vi "EchoSpacing.vi"() -> ()   [LabVIEW 2016]
uses:
  <vilib>/Analysis/3filter.llb/Filter Passband Type.ctl
  <vilib>/measure/NI_MABase.lvlib
  <vilib>/Analysis/NI_AALBase.lvlib
  <vilib>/measure/NI_MAPro.lvlib
panel:
  in  "Vertical Shift":dbl format="%#_13g"
  out "output waveform":waveform(dbl)(graph)
  out "Waveforms":waveform(dbl)[](graph)=[{"t0"=timestamp(0 s since 1904-01-01), "dt"=1e-06, "Y"=array[1000000 elements]}, {"t0"=timestamp(0 s since 1904-01-01), "dt"=1e-06, "Y"=array[1000000 elements]}]
  out "Waveform":waveform(dbl)(graph)={"t0"=timestamp(0 s since 1904-01-01), "dt"=1e-06, "Y"=array[1000000 elements]}
  in  "threshold":dbl format="%0.2f"
  in  "width":i32=3 min=3
  in  "low cutoff freq: fl":dbl=10.0 format="%0.4f"
  out "error":i32
  in  "order":i32=3
  out "total time":u32=122
  in  "frequency":dbl=40.0 format="%0.2p"
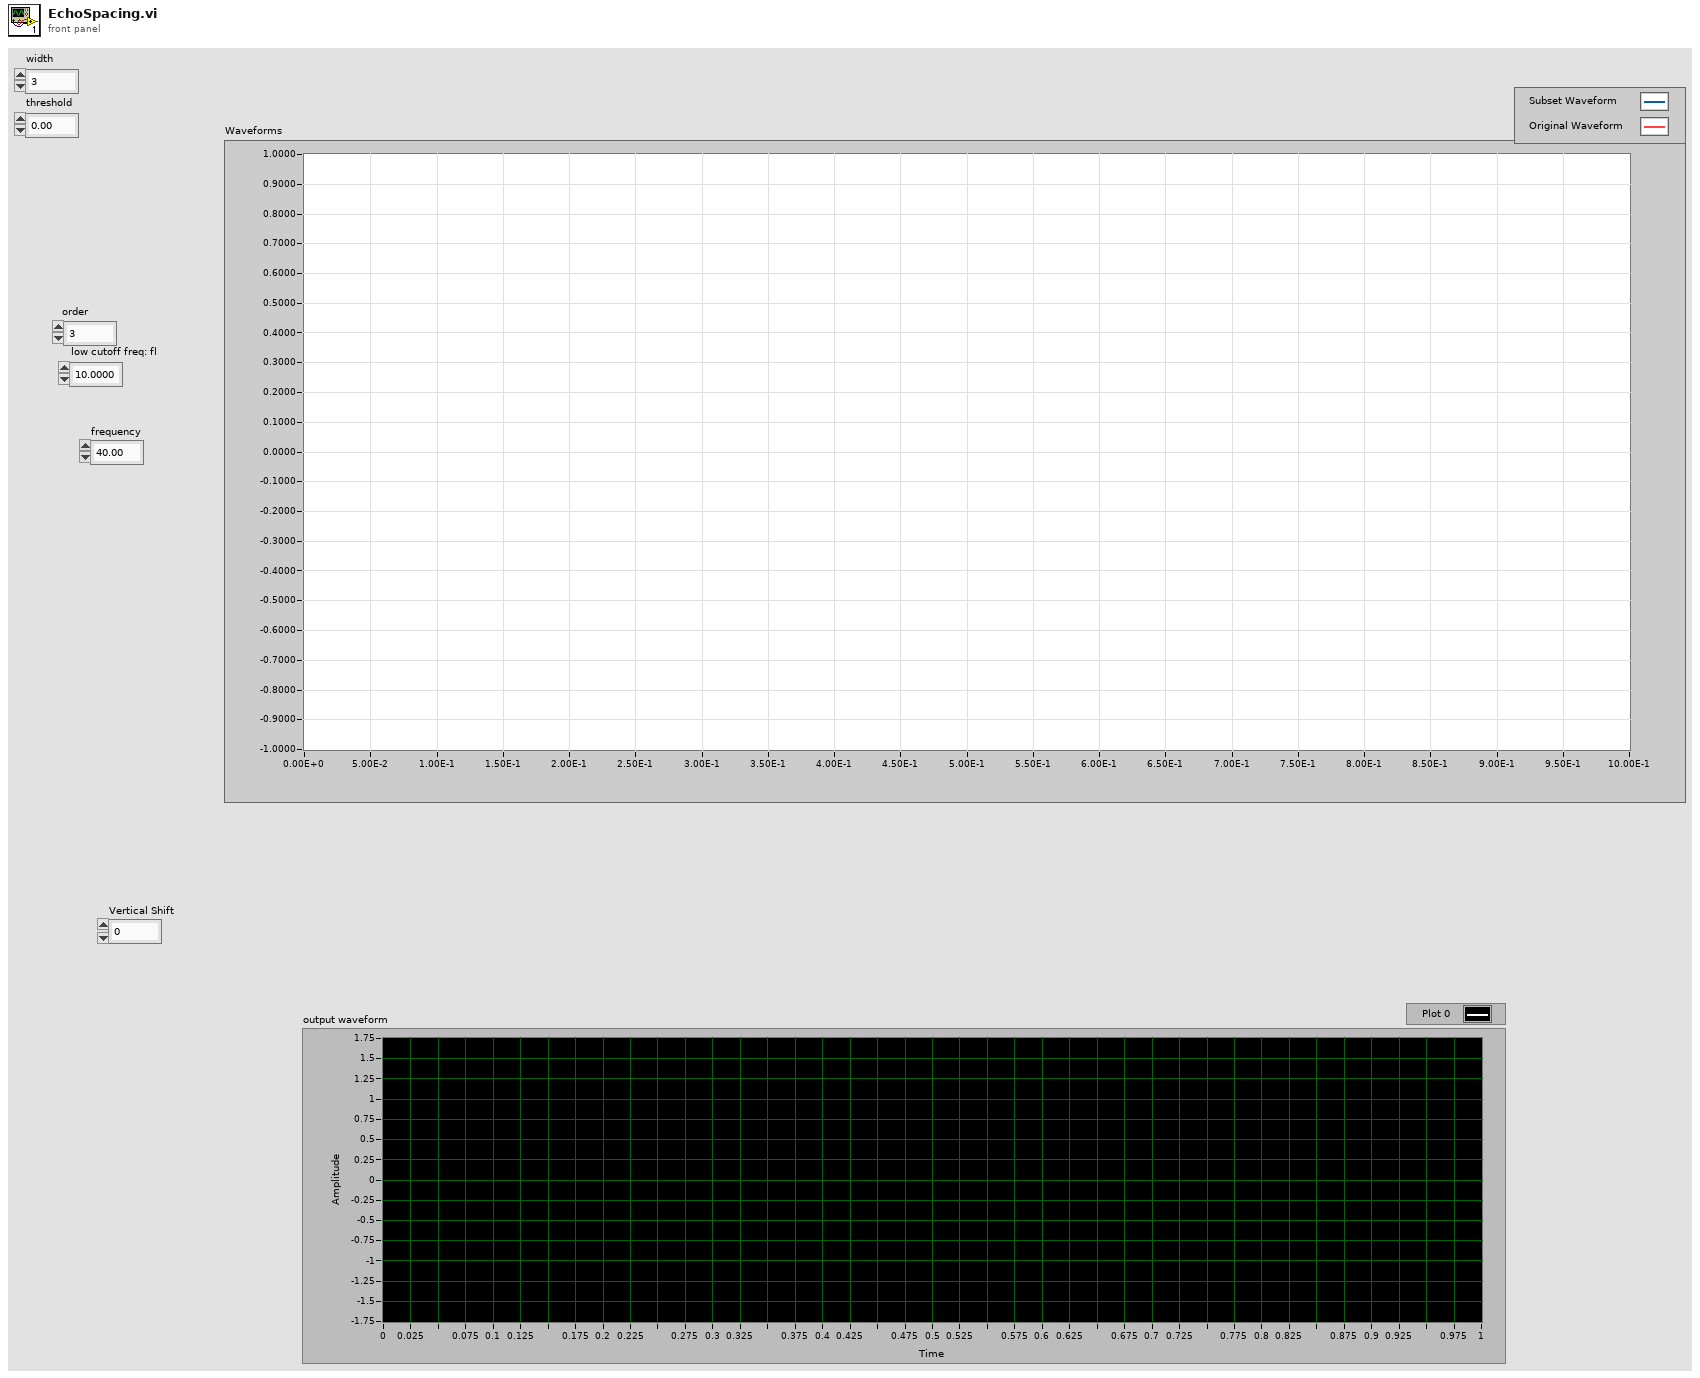
[diagram p1: front panel]
types:
  T1 = typedef "NI_AALBase.lvlib/Filter Passband Type.ctl" = enum32{"Lowpass", "Highpass", "Bandpass", "Bandstop"}
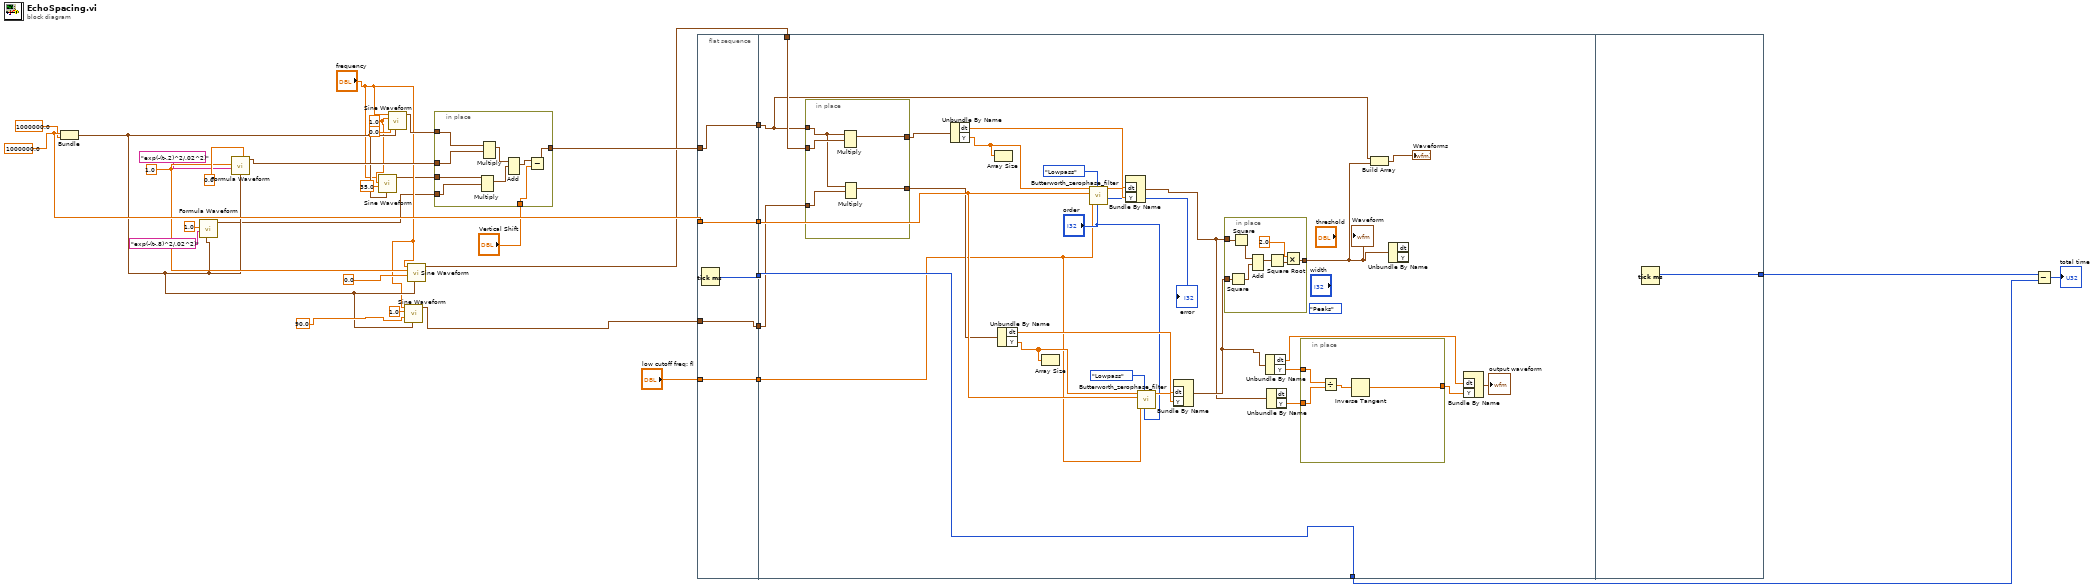
[diagram p0: block diagram]
diagram:
  w22 = 1.0 ("amplitude")
  w26 = 1000000.0
  w5 = 1.0 ("amplitude")
  n1 = Bundle(w26, 1000000.0) -> (w7:cluster{dbl, dbl})  [unwired: 1 in]
  n2 = call <vilib>:"Formula Waveform.vi"("sampling info"=w7, "formula"="exp(-(t-.8)^2/.02^2)", "amplitude"=1.0) -> ("signal out"=w2:waveform(dbl))  [unwired: 7 in, 1 out]
  n3 = call <vilib>:"Formula Waveform.vi"("offset"=0.0 ("phase"), "sampling info"=w7, "formula"="exp(-(t-.2)^2/.02^2)", "amplitude"=w22) -> ("signal out"=w8:waveform(dbl))  [unwired: 6 in, 1 out]
  n4 = call <vilib>:"Sine Waveform.vi"("sampling info"=w7, "phase"=35.0, "amplitude"=w5, "frequency"="frequency") -> ("signal out"=w3:waveform(dbl))  [unwired: 6 in, 1 out]
  n5 = call <vilib>:"Sine Waveform.vi"("sampling info"=w7, "phase"=0.0, "amplitude"=w5, "frequency"="frequency") -> ("signal out"=w27:waveform(dbl))  [unwired: 6 in, 1 out]
  n6 = call <vilib>:"Sine Waveform.vi"("sampling info"=w7, "phase"=90.0, "amplitude"=1.0, "frequency"="frequency") -> ("signal out"=w10:waveform(dbl))  [unwired: 6 in, 1 out]
  n7 = call <vilib>:"Sine Waveform.vi"("sampling info"=w7, "phase"=0.0, "amplitude"=w22, "frequency"="frequency") -> ("signal out"=w11:waveform(dbl))  [unwired: 6 in, 1 out]
  n8 = in-place {
    in-place-border: w27 -> [w41]
    in-place-border: w8 -> [w40]
    in-place-border: [w33] -> w17
    in-place-border: w3 -> [w39]
    in-place-border: w2 -> [w38]
    in-place-border: "Vertical Shift" -> [w34]
    n9 = Multiply(1:w38, 2:w39) -> (0:w36:waveform(dbl))  [unwired: 1 in, 1 out]
    n10 = Multiply(1:w40, 2:w41) -> (0:w37:waveform(dbl))  [unwired: 1 in, 1 out]
    n11 = Add(1:w36, 2:w37) -> (0:w35:waveform(dbl))  [unwired: 1 in, 1 out]
    n12 = Subtract(x=w35, y=w34) -> (x-y=w33:waveform(dbl))
  }
  n13 = flat-sequence {
    tunnel: [w46] -> w30
    tunnel: w26 -> [w45]
    tunnel: [w45] -> w25
    tunnel: [w44] -> w19
    tunnel: w10 -> [w44]
    tunnel: w17 -> [w43]
    tunnel: [w43] -> w16
    tunnel: "low cutoff freq: fl" -> [w42]
    tunnel: [w42] -> w14
    tunnel: [w73] -> w31
    tunnel: w30 -> [w73]
    tunnel: w25 -> [w63]
    tunnel: w19 -> [w60]
    tunnel: w11 -> [w57]
    tunnel: w16 -> [w54]
    tunnel: w14 -> [w58]
    tunnel: [w91] -> w32
    frame #0 {
      n14 = Tick Count (ms)() -> (millisecond timer value=w46:u32)
    }
    frame #1 {
      (unwired) enum32{"Peaks", "Valleys"}."Peaks" ("peaks/valleys")
      n15 = in-place {
        in-place-border: w54 -> [w80]
        in-place-border: w57 -> [w82]
        in-place-border: [w81] -> w61
        in-place-border: w60 -> [w79]
        in-place-border: [w78] -> w59
        n16 = Multiply(1:w82, 2:w80) -> (0:w81:waveform(dbl))  [unwired: 1 in, 1 out]
        n17 = Multiply(1:w79, 2:w80) -> (0:w78:waveform(dbl))  [unwired: 1 in, 1 out]
      }
      n18 = Unbundle By Name(w61) -> ("dt"=w68:dbl, "Y"=w69:dbl[])
      n19 = Array Size(array=w69) -> ()  [unwired: 1 out]
      n20 = Unbundle By Name(w59) -> ("dt"=w64:dbl, "Y"=w65:dbl[])
      n21 = Array Size(array=w65) -> ()  [unwired: 1 out]
      n22 = call "Butterworth_zerophase_filter.vi"("order"="order", "filter type"=Filter_Passband_Type."Lowpass", "low cutoff freq: fl"=w58, "sampling freq: fs"=w63, "X"=w69) -> ("error"=→"error":i32, "Filtered X"=w72:dbl[])  [unwired: 5 in]
      n23 = Bundle By Name("dt"=w68, "Y"=w72) -> (w52:waveform(dbl))  [unwired: 1 in]
      n24 = call "Butterworth_zerophase_filter.vi"("order"="order", "filter type"=Filter_Passband_Type."Lowpass", "low cutoff freq: fl"=w58, "sampling freq: fs"=w63, "X"=w65) -> ("Filtered X"=w67:dbl[])  [unwired: 5 in, 1 out]
      n25 = Bundle By Name("dt"=w64, "Y"=w67) -> (w53:waveform(dbl))  [unwired: 1 in]
      n26 = in-place {
        in-place-border: w52 -> [w90]
        in-place-border: w53 -> [w89]
        in-place-border: [w84] -> w56
        n27 = Square(x=w89) -> (x^2=w87:waveform(dbl))
        n28 = Square(x=w90) -> (x^2=w88:waveform(dbl))
        n29 = Add(1:w87, 2:w88) -> (0:w86:waveform(dbl))  [unwired: 1 in, 1 out]
        n30 = Square Root(x=w86) -> (sqrt(x)=w85:waveform(dbl))
        n31 = Multiply(x=2.0, y=w85) -> (x*y=w84:waveform(dbl))
      }
      "Waveform" <- w56
      n32 = Unbundle By Name(w53) -> ("dt"=w48:dbl, "Y"=w51:dbl[])
      n33 = Unbundle By Name(w52) -> ("Y"=w50:dbl[])  [unwired: 1 out]
      n34 = in-place {
        in-place-border: w51 -> [w77]
        in-place-border: w50 -> [w76]
        in-place-border: [w74] -> w49
        n35 = Divide(x=w77, y=w76) -> (x/y=w75:dbl[])
        n36 = Inverse Tangent(1:w75) -> (0:w74:dbl[])
      }
      n37 = Build Array(w54, w56) -> (→"Waveforms":waveform(dbl)[])
      n38 = Unbundle By Name(w56) -> ()  [unwired: 2 out]
      n39 = Bundle By Name("dt"=w48, "Y"=w49) -> (→"output waveform":waveform(dbl))  [unwired: 1 in]
    }
    frame #2 {
      n40 = Tick Count (ms)() -> (millisecond timer value=w91:u32)
    }
  }
  n41 = Subtract(x=w32, y=w31) -> (x-y=→"total time":u32)
